vi "TLB Native Dynamic Events ver 0.26e.vi"() -> ()   [LabVIEW 2018] (continued)
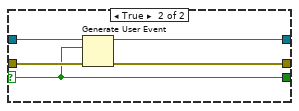
[diagram p2: hidden frame]
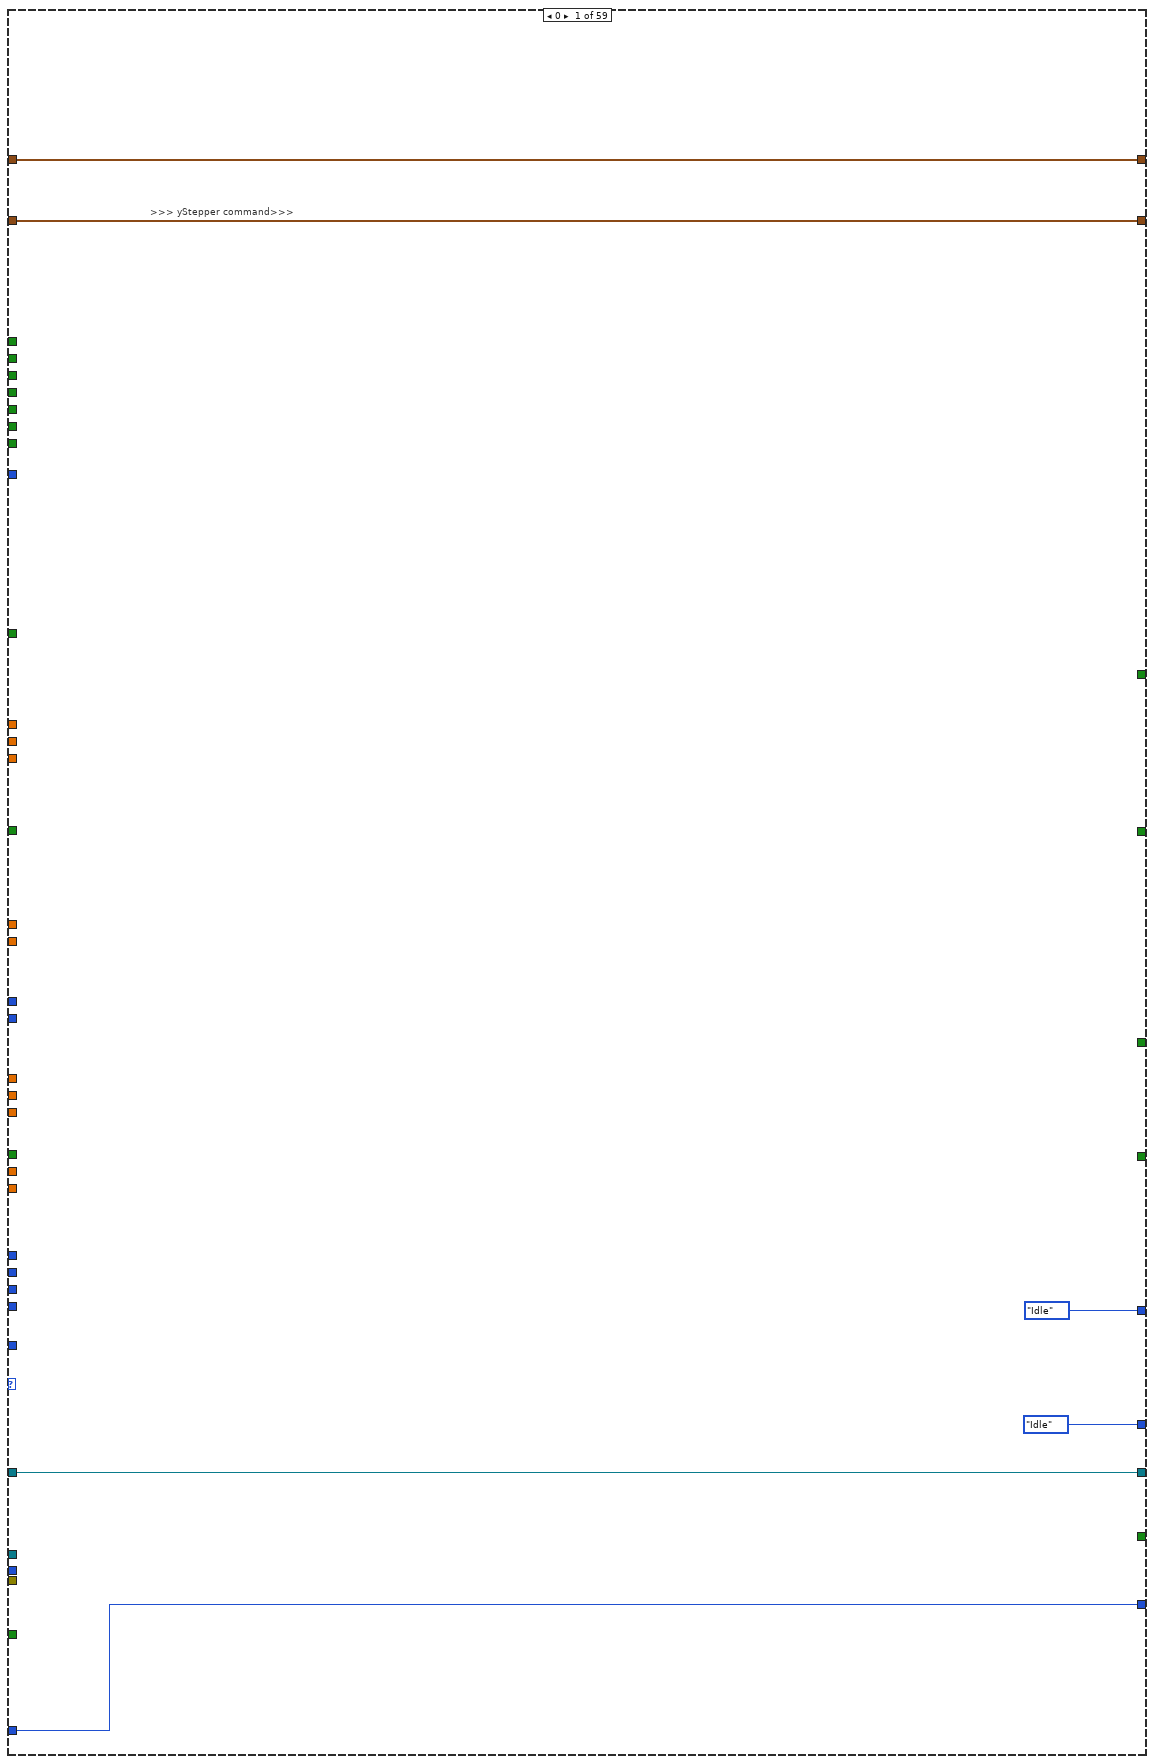
[diagram p5: hidden frame]
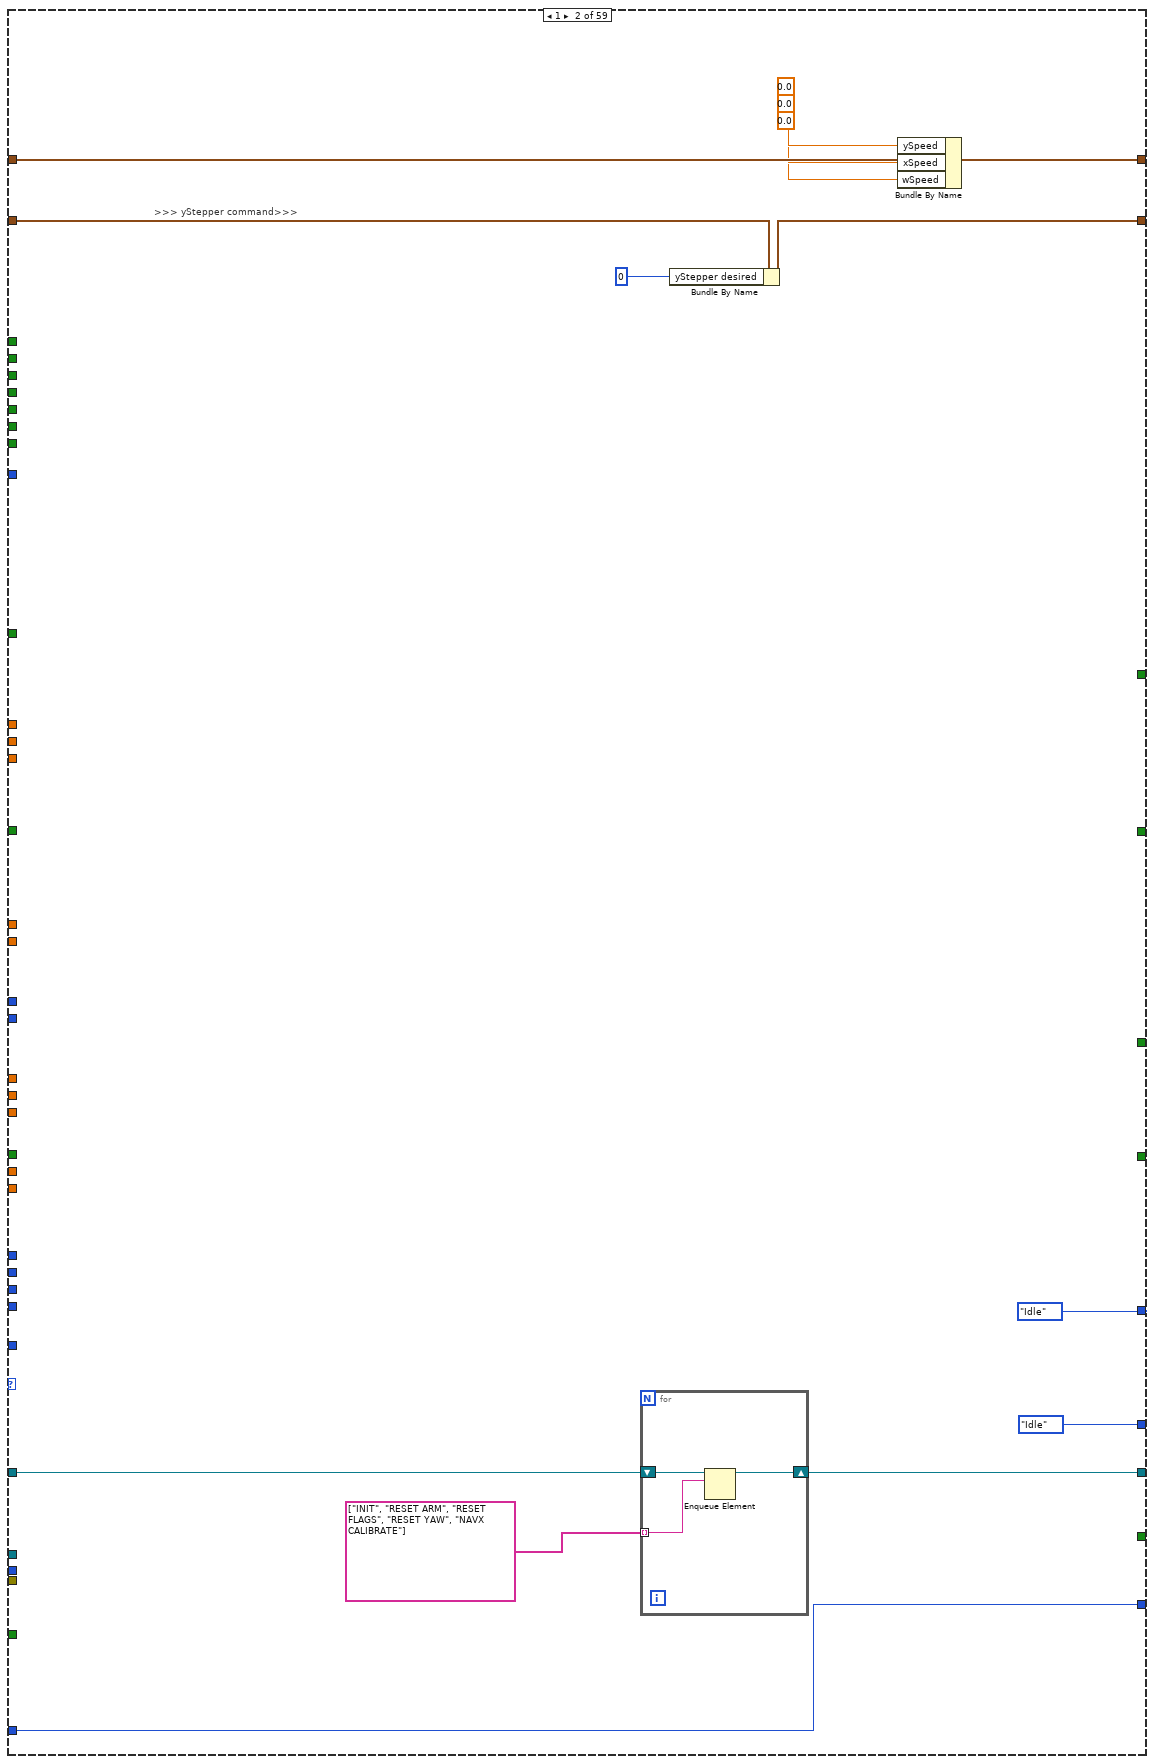
[diagram p6: hidden frame]
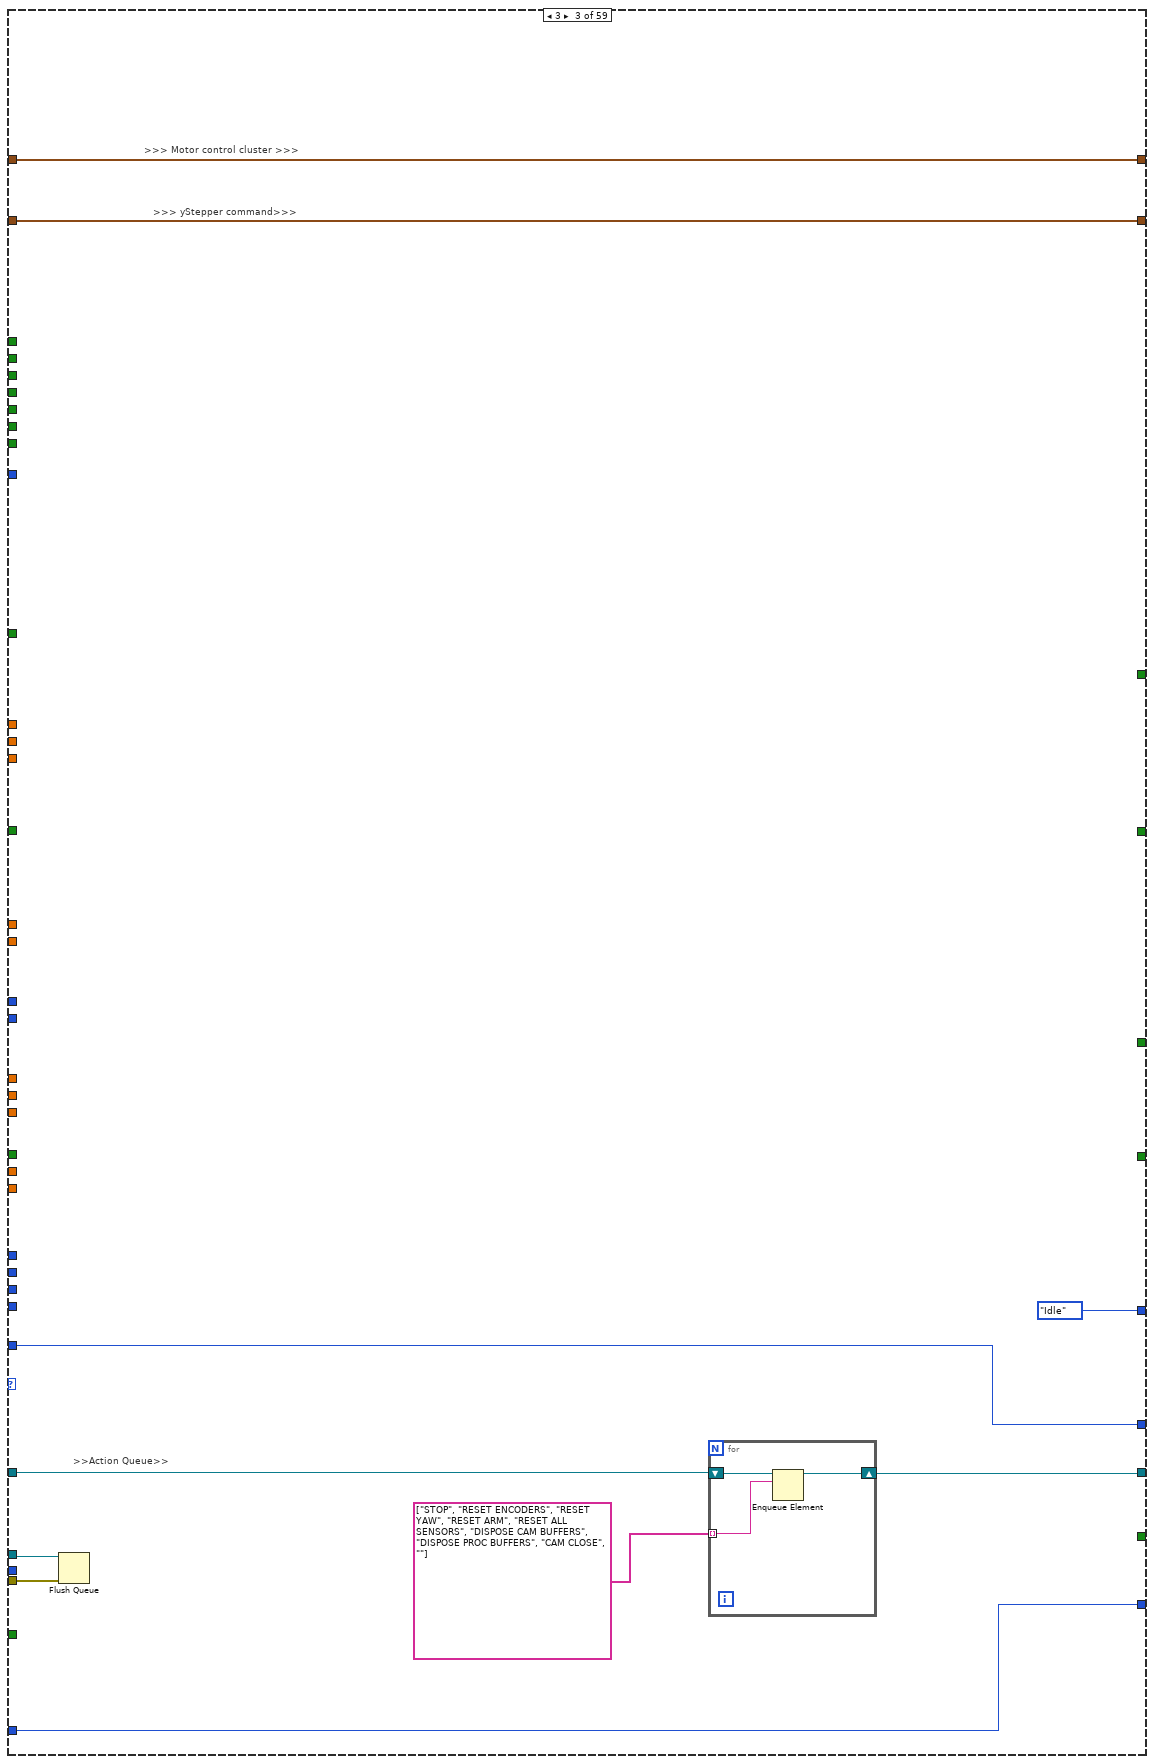
[diagram p7: hidden frame]
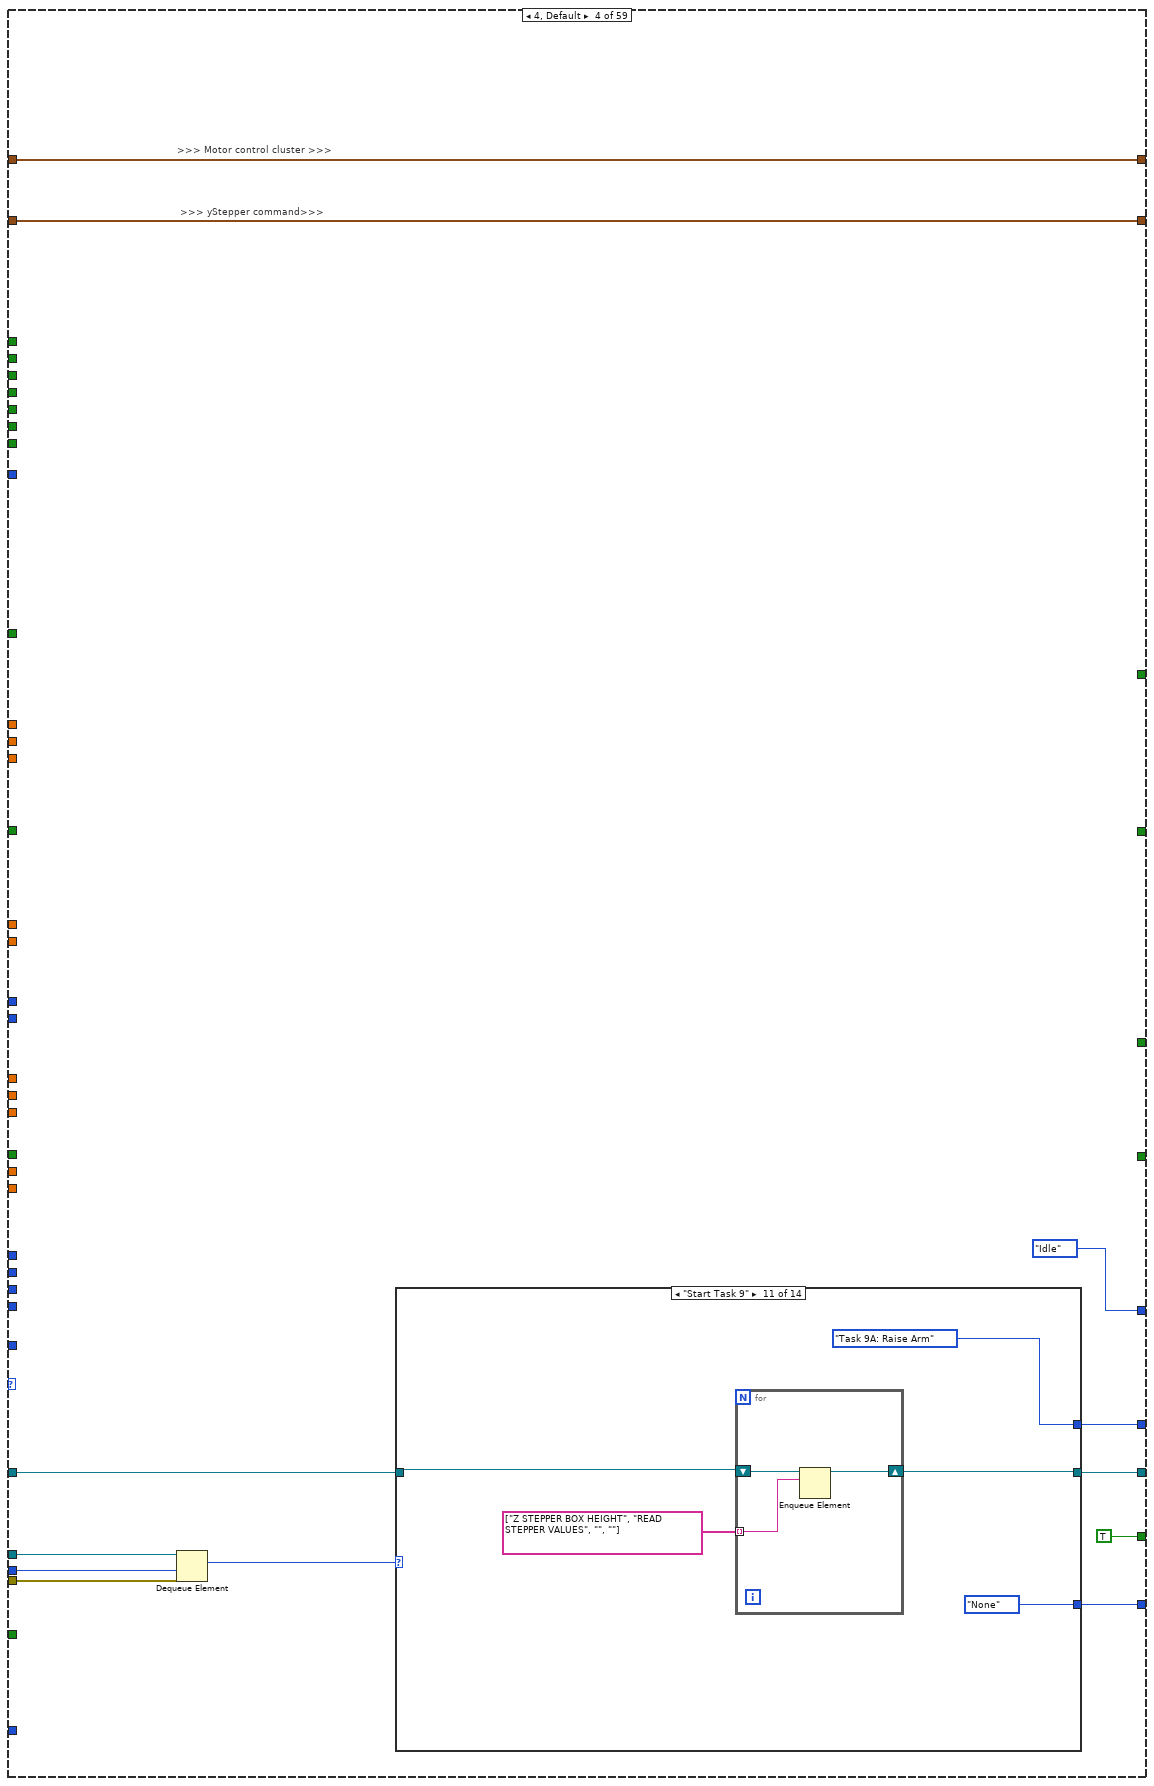
[diagram p8: hidden frame]
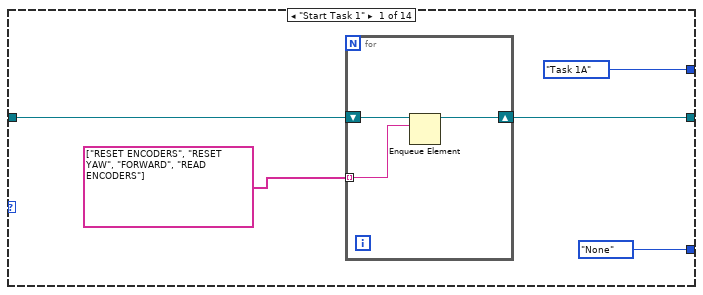
[diagram p9: hidden frame]
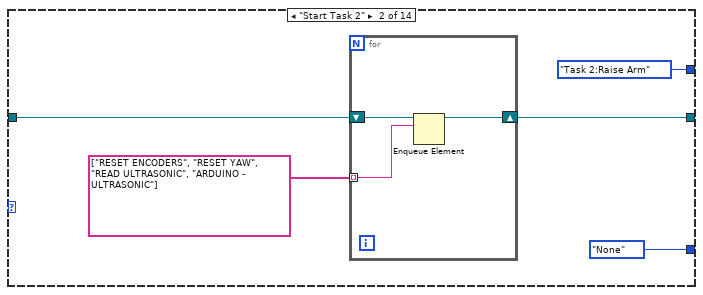
[diagram p10: hidden frame]
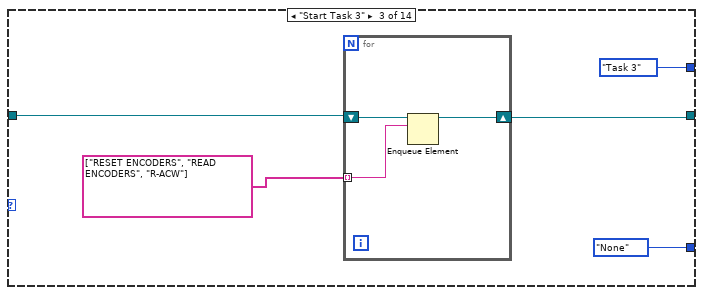
[diagram p11: hidden frame]
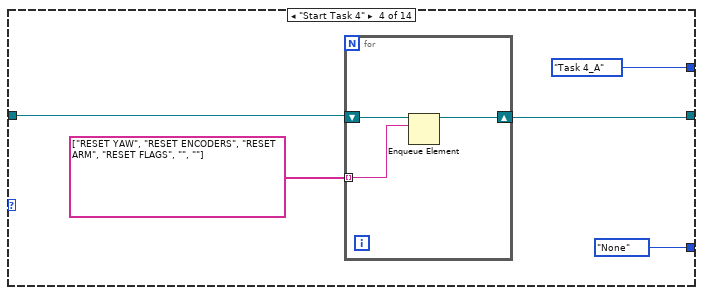
[diagram p12: hidden frame]
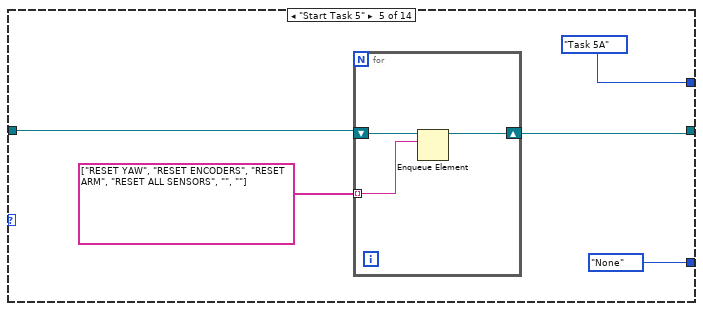
[diagram p13: hidden frame]
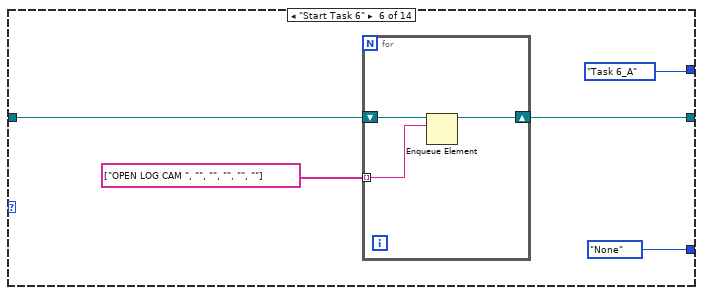
[diagram p14: hidden frame]
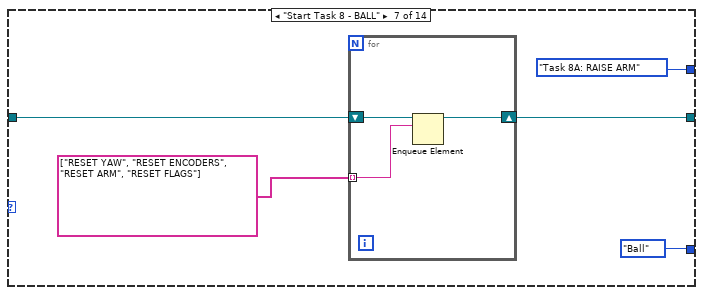
[diagram p15: hidden frame]
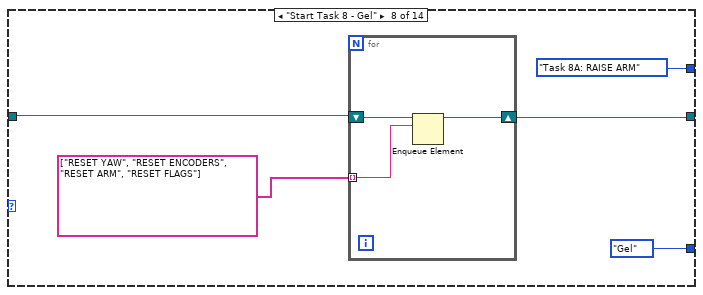
[diagram p16: hidden frame]
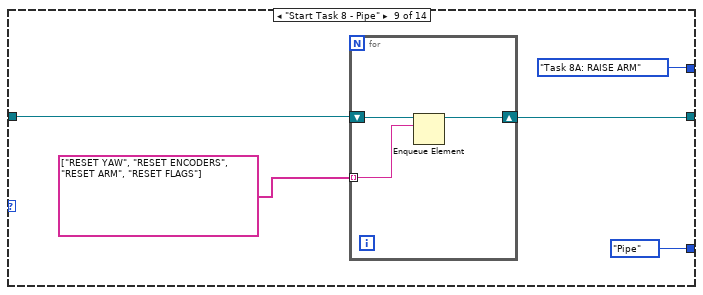
[diagram p17: hidden frame]
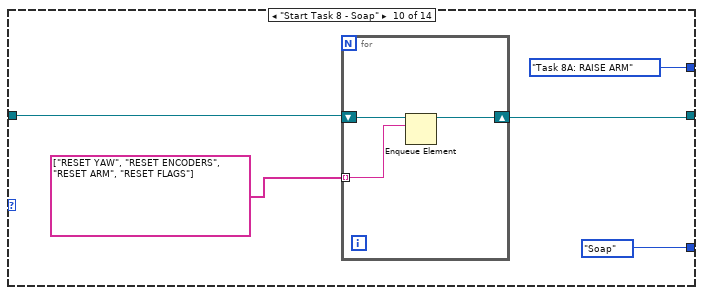
[diagram p18: hidden frame]
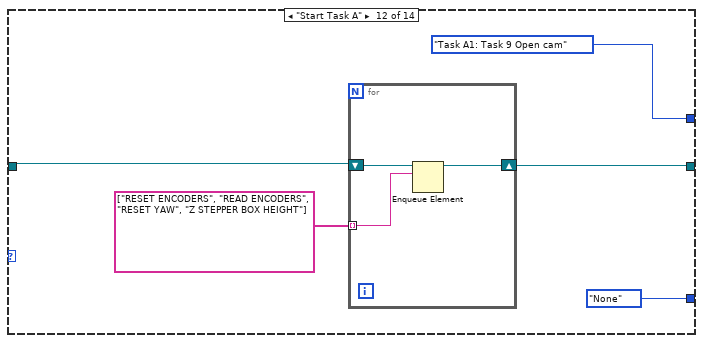
[diagram p19: hidden frame]
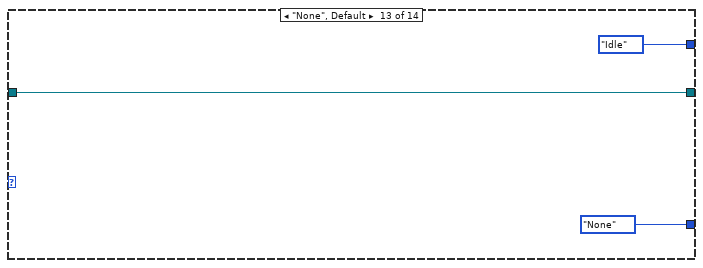
[diagram p20: hidden frame]
                  tunnel: [w2710 w2715] -> w2704
                  frame False {
                    n893 = for {
                      tunnel: string[] ["READ LINE SENSOR", "READ NAVX", "RIGHT", "READ ENCODERS"] ("element") -> [w2711] mode=indexing
                      shift-right: [w2713] -> w2710
                      shift-left: w2709 -> [w2712]
                      n894 = Enqueue Element(queue=w2712, element=w2711) -> (queue out=w2713:refnum<queue>)  [unwired: 2 in, 2 out]
                    }
                  }
                  frame True {
                    n895 = for {
                      shift-right: [w2718] -> w2715
                      shift-left: w2716 -> [w2719]
                      tunnel: string[] ["STOP", "RESET ENCODERS", "RESET YAW", "OPEN LIFE CAM", "SET TIMER 2", "RESET FLAGS"] -> [w2717] mode=indexing
                      n896 = Enqueue Element(queue=w2719, element=w2717) -> (queue out=w2718:refnum<queue>)  [unwired: 2 in, 2 out]
                    }
                  }
                }
                n897 = Or(x=w2699, y=w2698) -> (x .or. y?=w2697:bool)
                n898 = Select(t=State_Type_Definitions,_for_0.26g_versions_and_later_2."True Stop" ("Enum"), s=w2698, f=State_Type_Definitions,_for_0.26g_versions_and_later_2."PENIS 3" ("Enum")) -> (s? t:f=w2700:T18)
                n899 = Select(t=w2700, s=w2697, f=State_Type_Definitions,_for_0.26g_versions_and_later_2."PENIS 2" ("Enum")) -> (s? t:f=w2706:T18)
              }
              frame "Exit" {
                n900 = for {
                  shift-right: [w2726] -> w2723
                  shift-left: w2722 -> [w2727]
                  tunnel: string[] ["STOP", "RESET ENCODERS", "RESET YAW", "ARDUINO MODE 0"] -> [w2725] mode=indexing
                  n901 = Enqueue Element(queue=w2727, element=w2725) -> (queue out=w2726:refnum<queue>)  [unwired: 2 in, 2 out]
                }
              }
            }
          }
          frame 55 {
            # ">> Manual override >>"
            n902 = Dequeue Element(queue=w2736, timeout in ms (-1)=w2735, error in (no error)=w2734) -> (element=w2737:T10)  [unwired: 3 out]
            n903 = case shown="\"Start Task 1\", Default" w2737 {
              tunnel: [w2751 State_Type_Definitions,_for_0.26g_versions_and_later_2."True Stop" ("Enum")] -> w2729
              tunnel: [w2749 w2767] -> w2728
              tunnel: w2732 -> [w2748 w2764]
              tunnel: w2733 -> [w2742 _]
              tunnel: [State_Type_Definitions,_for_0.26g_versions_and_later_2."Idle" ("Enum") State_Type_Definitions,_for_0.26g_versions_and_later_2."Shutdown" ("Enum")] -> w2730
              tunnel: w2731 -> [w2741 _]
              frame "Start Task 1", Default {
                # ">> WIill proceed to part ii if not manual override >>"
                # ">>If ENABLE or Trigger is set to true>>"
                n904 = Or(x=w2741, y=w2742) -> (x .or. y?=w2743:bool)
                n905 = case shown="False" w2741 {
                  tunnel: [w2754 w2760] -> w2749
                  tunnel: w2748 -> [w2753 w2759]
                  frame False {
                    n906 = for {
                      shift-right: [w2756] -> w2754
                      shift-left: w2753 -> [w2757]
                      tunnel: string[] ["CAM ACQ", "START TIMER"] ("element") -> [w2755] mode=indexing
                      n907 = Enqueue Element(queue=w2757, element=w2755) -> (queue out=w2756:refnum<queue>)  [unwired: 2 in, 2 out]
                    }
                  }
                  frame True {
                    n908 = for {
                      shift-right: [w2762] -> w2760
                      shift-left: w2759 -> [w2763]
                      tunnel: string[] ["CLOSE CAM", "SET TIMER 5", "", "", "", ""] -> [w2761] mode=indexing
                      n909 = Enqueue Element(queue=w2763, element=w2761) -> (queue out=w2762:refnum<queue>)  [unwired: 2 in, 2 out]
                    }
                  }
                }
                n910 = Select(t=State_Type_Definitions,_for_0.26g_versions_and_later_2."True Stop" ("Enum"), s=w2742, f=State_Type_Definitions,_for_0.26g_versions_and_later_2."Task 9R: PROCESS COLOUR" ("Enum")) -> (s? t:f=w2745:T18)
                n911 = Select(t=w2745, s=w2743, f=State_Type_Definitions,_for_0.26g_versions_and_later_2."PENIS 3" ("Enum")) -> (s? t:f=w2751:T18)
              }
              frame "Exit" {
                n912 = for {
                  shift-right: [w2770] -> w2767
                  shift-left: w2764 -> [w2771]
                  tunnel: string[] ["STOP", "RESET ENCODERS", "RESET YAW", ""] -> [w2769] mode=indexing
                  n913 = Enqueue Element(queue=w2771, element=w2769) -> (queue out=w2770:refnum<queue>)  [unwired: 2 in, 2 out]
                }
              }
            }
          }
          frame 56 {
            # ">> Item Selection Bias >>"
            # ">>> Motor control cluster >>>"
            # ">>> yStepper command>>>"
            n914 = Dequeue Element(queue=w2777, timeout in ms (-1)=w2778, error in (no error)=w2779) -> (element=w2781:T10)  [unwired: 3 out]
            n915 = case shown="\"Start Task 1\", Default" w2781 {
              tunnel: w2775 -> [w2787 _]
              tunnel: [w2794 State_Type_Definitions,_for_0.26g_versions_and_later_2."True Stop" ("Enum")] -> w2773
              tunnel: w2780 -> [w2786 _]
              tunnel: w2776 -> [w2793 w2810]
              tunnel: [w2792 w2811] -> w2772
              tunnel: [State_Type_Definitions,_for_0.26g_versions_and_later_2."Idle" ("Enum") State_Type_Definitions,_for_0.26g_versions_and_later_2."Shutdown" ("Enum")] -> w2774
              frame "Start Task 1", Default {
                n916 = case shown="False" w2787 {
                  tunnel: w2793 -> [w2797 w2804]
                  tunnel: [w2798 w2803] -> w2792
                  frame False {
                    n917 = for {
                      tunnel: string[] ["START TIMER", "COLOUR PROCESSING", ""] ("element") -> [w2799] mode=indexing
                      shift-right: [w2801] -> w2798
                      shift-left: w2797 -> [w2800]
                      n918 = Enqueue Element(queue=w2800, element=w2799) -> (queue out=w2801:refnum<queue>)  [unwired: 2 in, 2 out]
                    }
                  }
                  frame True {
                    n919 = for {
                      shift-right: [w2806] -> w2803
                      shift-left: w2804 -> [w2807]
                      tunnel: string[] ["CLOSE CAM", "DISPOSE BUFFERS", "RESET ENCODERS", "RESET YAW", "RESET FLAGS", ""] -> [w2805] mode=indexing
                      n920 = Enqueue Element(queue=w2807, element=w2805) -> (queue out=w2806:refnum<queue>)  [unwired: 2 in, 2 out]
                    }
                  }
                }
                n921 = Or(x=w2787, y=w2786) -> (x .or. y?=w2785:bool)
                n922 = Select(t=State_Type_Definitions,_for_0.26g_versions_and_later_2."True Stop" ("Enum"), s=w2786, f=State_Type_Definitions,_for_0.26g_versions_and_later_2."True Stop" ("Enum")) -> (s? t:f=w2788:T18)
                n923 = Select(t=w2788, s=w2785, f=State_Type_Definitions,_for_0.26g_versions_and_later_2."Task 9R: PROCESS COLOUR" ("Enum")) -> (s? t:f=w2794:T18)
              }
              frame "Exit" {
                n924 = for {
                  shift-right: [w2814] -> w2811
                  shift-left: w2810 -> [w2815]
                  tunnel: string[] ["STOP", "RESET ENCODERS", "RESET YAW", "ARDUINO MODE 0"] -> [w2813] mode=indexing
                  n925 = Enqueue Element(queue=w2815, element=w2813) -> (queue out=w2814:refnum<queue>)  [unwired: 2 in, 2 out]
                }
              }
            }
          }
          frame 57 {
            # ">>> Motor control cluster >>>"
            # ">>> yStepper command>>>"
            # ">> Manual override >>"
            n926 = Dequeue Element(queue=w2827, timeout in ms (-1)=w2823, error in (no error)=w2826) -> (element=w2828:T10)  [unwired: 3 out]
            n927 = case shown="\"Start Task 1\", Default" w2828 {
              tunnel: [w2839 State_Type_Definitions,_for_0.26g_versions_and_later_2."True Stop" ("Enum")] -> w2821
              tunnel: [w2837 w2854] -> w2820
              tunnel: w2824 -> [w2836 _]
              tunnel: w2825 -> [w2830 _]
              tunnel: [State_Type_Definitions,_for_0.26g_versions_and_later_2."Idle" ("Enum") State_Type_Definitions,_for_0.26g_versions_and_later_2."Shutdown" ("Enum")] -> w2822
              tunnel: w2816 -> [w2829 _]
              frame "Start Task 1", Default {
                # ">> WIill proceed to part ii if not manual override >>"
                # ">>If ENABLE or Trigger is set to true>>"
                n928 = Or(x=w2829, y=w2830) -> (x .or. y?=w2831:bool)
                n929 = case shown="False" w2829 {
                  tunnel: [w2842 w2848] -> w2837
                  tunnel: w2836 -> [w2841 w2847]
                  frame False {
                    n930 = for {
                      shift-right: [w2844] -> w2842
                      shift-left: w2841 -> [w2845]
                      tunnel: string[] ["Task 9", ""] ("element") -> [w2843] mode=indexing
                      n931 = Enqueue Element(queue=w2845, element=w2843) -> (queue out=w2844:refnum<queue>)  [unwired: 2 in, 2 out]
                    }
                  }
                  frame True {
                    n932 = for {
                      shift-right: [w2850] -> w2848
                      shift-left: w2847 -> [w2851]
                      tunnel: string[] ["ARDUINO - ULTRASONIC", "READ NAVX", "RESET FLAGS", "", "", ""] -> [w2849] mode=indexing
                      n933 = Enqueue Element(queue=w2851, element=w2849) -> (queue out=w2850:refnum<queue>)  [unwired: 2 in, 2 out]
                    }
                  }
                }
                n934 = Select(t=State_Type_Definitions,_for_0.26g_versions_and_later_2."True Stop" ("Enum"), s=w2830, f=State_Type_Definitions,_for_0.26g_versions_and_later_2."True Stop" ("Enum")) -> (s? t:f=w2833:T18)
                n935 = Select(t=w2833, s=w2831, f=State_Type_Definitions,_for_0.26g_versions_and_later_2."Task A1: Task 9 Open cam" ("Enum")) -> (s? t:f=w2839:T18)
              }
              frame "Exit" {
                n936 = for {
                  shift-right: [w2857] -> w2854
                  shift-left: _ -> [w2858]
                  tunnel: string[] ["STOP", "RESET ENCODERS", "RESET YAW", ""] -> [w2856] mode=indexing
                  n937 = Enqueue Element(queue=w2858, element=w2856) -> (queue out=w2857:refnum<queue>)  [unwired: 2 in, 2 out]
                }
              }
            }
          }
          frame 58 {
            # ">>> Motor control cluster >>>"
            # ">>> yStepper command>>>"
            n938 = Dequeue Element(queue=w2872, timeout in ms (-1)=w2871, error in (no error)=w2870) -> (element=w2874:T10)  [unwired: 3 out]
            n939 = In Range and Coerce(upper limit=65.0, x=w2864, lower limit=58.0) -> (In Range?=w2861:bool)  [unwired: 1 out]
            n940 = case shown="\"Start Task 1\", Default" w2874 {
              tunnel: w2865 -> [w2877 _]
              tunnel: [w2885 State_Type_Definitions,_for_0.26g_versions_and_later_2."True Stop" ("Enum")] -> w2867
              tunnel: w2873 -> [w2883 w2901]
              tunnel: [w2882 w2900] -> w2866
              tunnel: [State_Type_Definitions,_for_0.26g_versions_and_later_2."Idle" ("Enum") State_Type_Definitions,_for_0.26g_versions_and_later_2."Shutdown" ("Enum")] -> w2868
              tunnel: w2861 -> [w2875 _]
              frame "Start Task 1", Default {
                n941 = Or(x=w2875, y=w2877) -> (x .or. y?=w2876:bool)
                n942 = case shown="True" w2875 {
                  tunnel: w2883 -> [w2888 w2894]
                  tunnel: [w2887 w2892] -> w2882
                  frame False {
                    n943 = for {
                      shift-right: [w2890] -> w2887
                      shift-left: w2888 -> [w2891]
                      tunnel: string[] ["READ NAVX", "R-CW", "READ ULTRASONIC"] ("element") -> [w2889] mode=indexing
                      n944 = Enqueue Element(queue=w2891, element=w2889) -> (queue out=w2890:refnum<queue>)  [unwired: 2 in, 2 out]
                    }
                  }
                  frame True {
                    n945 = for {
                      shift-right: [w2896] -> w2892
                      shift-left: w2894 -> [w2897]
                      tunnel: string[] ["STOP", "RESET ENCODERS", "RESET YAW", "READ IR", "ARDUINO - ULTRASONIC"] -> [w2895] mode=indexing
                      n946 = Enqueue Element(queue=w2897, element=w2895) -> (queue out=w2896:refnum<queue>)  [unwired: 2 in, 2 out]
                    }
                  }
                }
                n947 = Select(t=State_Type_Definitions,_for_0.26g_versions_and_later_2."True Stop" ("Enum"), s=w2877, f=State_Type_Definitions,_for_0.26g_versions_and_later_2."Task A3: Task 9 Set Timer") -> (s? t:f=w2879:T18)
                n948 = Select(t=w2879, s=w2876, f=State_Type_Definitions,_for_0.26g_versions_and_later_2."Task A2: Task 9 Move Arm" ("Enum")) -> (s? t:f=w2885:T18)
              }
              frame "Exit" {
                n949 = for {
                  shift-right: [w2904] -> w2900
                  shift-left: w2901 -> [w2905]
                  tunnel: string[] ["STOP", "RESET ENCODERS", "RESET YAW", ""] -> [w2903] mode=indexing
                  n950 = Enqueue Element(queue=w2905, element=w2903) -> (queue out=w2904:refnum<queue>)  [unwired: 2 in, 2 out]
                }
              }
            }
          }
          frame 59 {
            (unwired) 50.0 ("y")
            (unwired) 15.0 ("y")
            # ">> Item Selection Bias >>"
            # ">> Wall detected >>"
            # ">> Manual override >>"
            # ">>> Motor control cluster >>>"
            # ">>Table or wall detectected>>"
            # ">>Action Queue>>"
            # ">>> yStepper command>>>"
            n951 = Dequeue Element(queue=w2921, timeout in ms (-1)=w2920, error in (no error)=w2919) -> (element=w2922:T10)  [unwired: 3 out]
            n952 = Less?(x=w2908, y=100.0) -> (x < y?=w2909:bool)
            n953 = Not Equal To 0?(x=w2908) -> (x != 0?=w2907:bool)
            n954 = And(x=w2907, y=w2909) -> (x .and. y?=w2906:bool)
            n955 = case shown="\"Start Task 1\", Default" w2922 {
              tunnel: w2917 -> [w2923 _]
              tunnel: [w2933 State_Type_Definitions,_for_0.26g_versions_and_later_2."True Stop" ("Enum")] -> w2914
              tunnel: w2918 -> [w2931 w2949]
              tunnel: [w2930 w2948] -> w2913
              tunnel: [State_Type_Definitions,_for_0.26g_versions_and_later_2."Idle" ("Enum") State_Type_Definitions,_for_0.26g_versions_and_later_2."Shutdown" ("Enum")] -> w2916
              tunnel: w2906 -> [w2924 _]
              frame "Start Task 1", Default {
                n956 = Or(x=w2923, y=w2924) -> (x .or. y?=w2925:bool)
                n957 = case shown="False" w2924 {
                  tunnel: w2931 -> [w2936 w2942]
                  tunnel: [w2935 w2940] -> w2930
                  frame False {
                    n958 = for {
                      shift-right: [w2938] -> w2935
                      shift-left: w2936 -> [w2939]
                      tunnel: string[] ["READ IR", "FORWARD - IR ASSIST", "READ ULTRASONIC"] ("element") -> [w2937] mode=indexing
                      n959 = Enqueue Element(queue=w2939, element=w2937) -> (queue out=w2938:refnum<queue>)  [unwired: 2 in, 2 out]
                    }
                  }
                  frame True {
                    n960 = for {
                      shift-right: [w2944] -> w2940
                      shift-left: w2942 -> [w2945]
                      tunnel: string[] ["STOP", "RESET ENCODERS", "RESET YAW", ""] -> [w2943] mode=indexing
                      n961 = Enqueue Element(queue=w2945, element=w2943) -> (queue out=w2944:refnum<queue>)  [unwired: 2 in, 2 out]
                    }
                  }
                }
                n962 = Select(t=State_Type_Definitions,_for_0.26g_versions_and_later_2."True Stop" ("Enum"), s=w2923, f=State_Type_Definitions,_for_0.26g_versions_and_later_2."Task A4: Tasl 9 Capture images") -> (s? t:f=w2927:T18)
                n963 = Select(t=w2927, s=w2925, f=State_Type_Definitions,_for_0.26g_versions_and_later_2."Task A3: Task 9 Set Timer" ("Enum")) -> (s? t:f=w2933:T18)
              }
              frame "Exit" {
                n964 = for {
                  shift-right: [w2952] -> w2948
                  shift-left: w2949 -> [w2953]
                  tunnel: string[] ["STOP", "RESET ENCODERS", "RESET YAW", ""] -> [w2951] mode=indexing
                  n965 = Enqueue Element(queue=w2953, element=w2951) -> (queue out=w2952:refnum<queue>)  [unwired: 2 in, 2 out]
                }
              }
            }
          }
          frame 60 {
            # ">>> Motor control cluster >>>"
            # ">>> yStepper command>>>"
            # ">> Item Selection Bias >>"
            n966 = Less?(x=w2957, y=-40.0) -> (x < y?=w2955:bool)
            n967 = Dequeue Element(queue=w2963, timeout in ms (-1)=w2962, error in (no error)=w2961) -> (element=w2965:T10)  [unwired: 3 out]
            n968 = case shown="\"Start Task 1\", Default" w2965 {
              tunnel: w2955 -> [w2971 _]
              tunnel: [w2978 State_Type_Definitions,_for_0.26g_versions_and_later_2."True Stop" ("Enum")] -> w2959
              tunnel: w2960 -> [w2970 _]
              tunnel: w2964 -> [w2977 w2994]
              tunnel: [w2976 w2995] -> w2954
              tunnel: [State_Type_Definitions,_for_0.26g_versions_and_later_2."Idle" ("Enum") State_Type_Definitions,_for_0.26g_versions_and_later_2."Shutdown" ("Enum")] -> w2958
              frame "Start Task 1", Default {
                n969 = case shown="True" w2971 {
                  tunnel: w2977 -> [w2981 w2988]
                  tunnel: [w2982 w2987] -> w2976
                  frame False {
                    n970 = for {
                      tunnel: string[] ["READ ENCODERS", "R-CW"] ("element") -> [w2983] mode=indexing
                      shift-right: [w2985] -> w2982
                      shift-left: w2981 -> [w2984]
                      n971 = Enqueue Element(queue=w2984, element=w2983) -> (queue out=w2985:refnum<queue>)  [unwired: 2 in, 2 out]
                    }
                  }
                  frame True {
                    n972 = for {
                      shift-right: [w2990] -> w2987
                      shift-left: w2988 -> [w2991]
                      tunnel: string[] ["STOP", "RESET ENCODERS", "RESET FLAGS", "RESET YAW", "READ IR", ""] -> [w2989] mode=indexing
                      n973 = Enqueue Element(queue=w2991, element=w2989) -> (queue out=w2990:refnum<queue>)  [unwired: 2 in, 2 out]
                    }
                  }
                }
                n974 = Or(x=w2971, y=w2970) -> (x .or. y?=w2969:bool)
                n975 = Select(t=State_Type_Definitions,_for_0.26g_versions_and_later_2."True Stop" ("Enum"), s=w2970, f=State_Type_Definitions,_for_0.26g_versions_and_later_2."Task A3: Task 9 Set Timer" ("Enum")) -> (s? t:f=w2972:T18)
                n976 = Select(t=w2972, s=w2969, f=State_Type_Definitions,_for_0.26g_versions_and_later_2."Task A4: Tasl 9 Capture images" ("Enum")) -> (s? t:f=w2978:T18)
              }
              frame "Exit" {
                n977 = for {
                  shift-right: [w2998] -> w2995
                  shift-left: w2994 -> [w2999]
                  tunnel: string[] ["STOP", "RESET ENCODERS", "RESET YAW", "ARDUINO MODE 0"] -> [w2997] mode=indexing
                  n978 = Enqueue Element(queue=w2999, element=w2997) -> (queue out=w2998:refnum<queue>)  [unwired: 2 in, 2 out]
                }
              }
            }
          }
        }
        "Object Detection" <- w336
        "Ultrasonic sensors" <- w359
        "Encoder values" <- w348
        "Stepper position values" <- w332
        "NAVX Values" <- w330
        "IR Sensors" <- w322
        "Line sensors" <- w317
        "Time cluster" <- w328
        "Box Colour Detection" <- w310
      }
    }
    "Object recognition mode" <- w234
    "Front Ultrasonic obstruct" <- w231
    "Front IR obstruct" <- w230
    "Table IR obstruct" <- w229
    "Same colour?" <- w224
    n979 = local write "Green LED"(w244) -> ()
  }
  n980 = while {
    stop <- w3910 stop-if-true
    n981 = call "MOTOR CONTROL WITH PID AE.vi"("AE Mode"=MOTOR_CONTROL_WITH_PID_AE_DATA_MODE_TYPE_DEF."Read from AE") -> ("Speed & distance"=→"Speed & distance":T15)  [unwired: 3 in]
    n982 = call "FGV Stop.vi"("Init/Read/Write State"=States_for_Action_Engine."Read") -> ("Output node"=w3910:bool)  [unwired: 2 in, 1 out]
    n983 = Wait (ms)(milliseconds to wait=u32 5) -> ()  [unwired: 1 out]
  }
  n984 = call <vilib>:"DIO Close.vi"("error in (no error)"=w23, "DIO Info In"=w26) -> ()  [unwired: 9 in, 1 out]
  n985 = call <vilib>:"DIO Close.vi"("error in (no error)"=w33, "DIO Info In"=w35) -> ()  [unwired: 9 in, 1 out]
  n986 = call <vilib>:"NavX Close.vi"("error in (no error)"=w10, "NavX Info In"=w9) -> ()  [unwired: 9 in, 1 out]
  n987 = call <vilib>:"DIO Close.vi"("error in (no error)"=w28, "DIO Info In"=w30) -> ()  [unwired: 9 in, 1 out]
  n988 = call <vilib>:"DIO Close.vi"("error in (no error)"=w17, "DIO Info In"=w18) -> ()  [unwired: 9 in, 1 out]
  n989 = call <vilib>:"DIO Close.vi"("error in (no error)"=w12, "DIO Info In"=w13) -> ()  [unwired: 9 in, 1 out]
  n990 = Merge Errors "Merge Errors"(w63, w62) -> (w45:errorcluster)
  n991 = Merge Errors(w49, w45) -> (w44:errorcluster)
  n992 = Destroy User Event(user event=w67, error in=w44) -> ()  [unwired: 1 out]
  n993 = Release Queue(queue=w40, error in (no error)=w44) -> (error out=→"Queue Errors":errorcluster)  [unwired: 1 in, 2 out]
  n994 = Release Queue(queue=w57, error in (no error)=w44) -> ()  [unwired: 1 in, 3 out]
  n995 = Destroy User Event(user event=w66, error in=w44) -> ()  [unwired: 1 out]
  n996 = Unregister For Events(event registration refnum=w58, error in=w44) -> ()  [unwired: 1 out]
